vi "Load Default Modes v2.vi"(9 "SLM Param In":T1={"Error"={"status"=FALSE, "code"=0, "source"=""}, "References"={"Main VI"=refnum, "SLM VI"=refnum}, "Directories"={"Root Directory"=path "C:/Documents and Settings/tg273/My Documents/LabView VIs/Yale SLM/Yale v2/Mode Matrices", "Output Directory"=path "C:/Documents and Settings/tg273/My Documents/LabView VIs/Yale SLM/Yale v2/Mode Matrices"}, "Holo size"=504, "X pos"=-3, "Y pos"=-40, "Mode Coeffs"=[[2.0, 0.0], [3.0, 18.0], [4.0, 0.0], [11.0, 0.0], [22.0, 0.0], [37.0, 0.0], [5.0, 0.0], [6.0, 0.0], [7.0, 0.0], [8.0, 0.0], [9.0, 0.0], [10.0, 0.0]], "Wrap Value"=197, "Lambda (nm)"=750.0, "NA"=1.4, "Base Name"="", "Win Num"=2, "SLM SN"="0600535", "Holo Image Name"="0600535", "Matrix Name"="Unit Matrix.csv", "Mode Matrix"=array36x36[1296 elements], "Flatness"=array600x792[475200 elements], "STED Phase"=array504x504[254016 elements], "Ab Corr"=array504x504[254016 elements], "Holo Image"="remote image 00000000298188F4", "Holo Position"={-3.0, -40.0, 3840.0, 504.0}, "Apply Flatness\ncorr.?"=TRUE, "Max Wavelength (nm)"=750.0, "Min Wavelength (nm)"=750.0, "Vortex Rotation"=-3, "Top Hat Radius"=1.4, "SLM ID Num"="0600535", "Max Zernike Modes"=-3, "Screen Width"=2, "Ab Corr VI"={"AC VI Ref"=refnum, "# Modes"=2, "Mode Array"=[[4.0, 0.0, 0.0, 1.0, 0.0], [11.0, 0.75, 0.0, 1.0, 0.0], [22.0, 0.1, 0.0, 1.0, 0.0], [37.0, 0.0, 0.0, 1.0, 0.0], [7.0, 0.15, 0.0, 1.0, 0.0], [8.0, 0.1, 0.0, 1.0, 0.0], [5.0, 0.05, 0.0, 1.0, 0.0], [6.0, 0.0, 0.0, 1.0, 0.0], [9.0, 0.0, 0.0, 1.0, 0.0], [10.0, 0.0, 0.0, 1.0, 0.0], [2.0, 0.0, 0.0, 1.0, 0.0], [3.0, -18.3, 0.0, 1.0, 0.0]], "Apply Corr?"=TRUE, "Step Size"=0.3, "# Steps  "=11, "Resolution"=0.2, "FOV (um)"=12.0, "Metric Images"=[], "Metric Values"=[], "S"=[120.26, 128.5, 131.1, 136.15, 138.3, 148.05, 149.99, 150.02, 147.88, 152.65, 152.69, 150.56, 144.92, 143.08, 146.19, 140.15, 134.69, 125.47, 117.35, 108.32], "I"=[], "M"=[], "Coeff Steps"=[120.26, 128.5, 131.1, 136.15, 138.3, 148.05, 149.99, 150.02, 147.88, 152.65, 152.69, 150.56, 144.92, 143.08, 146.19, 140.15, 134.69, 125.47, 117.35, 108.32], "Mode Loop"={"Mode"=0, "Metric"=0, "Loop Index"=0}}} {"Vortex Rotation" format="%#_3g"; "Min Wavelength (nm)" format="%#_3g"; "Max Wavelength (nm)" format="%#_3g"; "Mode Matrix" format="%0.3f"; "Wrap Value" format="%#_3g"}) -> (1 "SLM Param Out":T1={"Error"={"status"=FALSE, "code"=0, "source"=""}, "References"={"Main VI"=refnum, "SLM VI"=refnum}, "Directories"={"Root Directory"=path "C:/Documents and Settings/tg273/My Documents/LabView VIs/Yale SLM/Yale v2/Mode Matrices", "Output Directory"=path "C:/Documents and Settings/tg273/My Documents/LabView VIs/Yale SLM/Yale v2/Mode Matrices"}, "Holo size"=504, "X pos"=-3, "Y pos"=-40, "Mode Coeffs"=[[2.0, 0.0], [3.0, 18.0], [4.0, 0.0], [11.0, 0.0], [22.0, 0.0], [37.0, 0.0], [5.0, 0.0], [6.0, 0.0], [7.0, 0.0], [8.0, 0.0], [9.0, 0.0], [10.0, 0.0]], "Wrap Value"=197, "Lambda (nm)"=750.0, "NA"=1.4, "Base Name"="", "Win Num"=2, "SLM SN"="0600535", "Holo Image Name"="0600535", "Matrix Name"="Unit Matrix.csv", "Mode Matrix"=array36x36[1296 elements], "Flatness"=array600x792[475200 elements], "STED Phase"=array504x504[254016 elements], "Ab Corr"=array504x504[254016 elements], "Holo Image"="remote image 00000000298188F4", "Holo Position"={-3.0, -40.0, 3840.0, 504.0}, "Apply Flatness\ncorr.?"=TRUE, "Max Wavelength (nm)"=750.0, "Min Wavelength (nm)"=750.0, "Vortex Rotation"=-3, "Top Hat Radius"=1.4, "SLM ID Num"="0600535", "Max Zernike Modes"=-3, "Screen Width"=2, "Ab Corr VI"={"AC VI Ref"=refnum, "# Modes"=2, "Mode Array"=[[4.0, 0.0, 0.0, 1.0, 0.0], [11.0, 0.75, 0.0, 1.0, 0.0], [22.0, 0.1, 0.0, 1.0, 0.0], [37.0, 0.0, 0.0, 1.0, 0.0], [7.0, 0.15, 0.0, 1.0, 0.0], [8.0, 0.1, 0.0, 1.0, 0.0], [5.0, 0.05, 0.0, 1.0, 0.0], [6.0, 0.0, 0.0, 1.0, 0.0], [9.0, 0.0, 0.0, 1.0, 0.0], [10.0, 0.0, 0.0, 1.0, 0.0], [2.0, 0.0, 0.0, 1.0, 0.0], [3.0, -18.3, 0.0, 1.0, 0.0]], "Apply Corr?"=TRUE, "Step Size"=0.3, "# Steps  "=11, "Resolution"=0.2, "FOV (um)"=12.0, "Metric Images"=[], "Metric Values"=[], "S"=[120.26, 128.5, 131.1, 136.15, 138.3, 148.05, 149.99, 150.02, 147.88, 152.65, 152.69, 150.56, 144.92, 143.08, 146.19, 140.15, 134.69, 125.47, 117.35, 108.32], "I"=[], "M"=[], "Coeff Steps"=[120.26, 128.5, 131.1, 136.15, 138.3, 148.05, 149.99, 150.02, 147.88, 152.65, 152.69, 150.56, 144.92, 143.08, 146.19, 140.15, 134.69, 125.47, 117.35, 108.32], "Mode Loop"={"Mode"=0, "Metric"=0, "Loop Index"=0}}} {"Vortex Rotation" format="%#_3g"; "Min Wavelength (nm)" format="%#_3g"; "Max Wavelength (nm)" format="%#_3g"; "Mode Matrix" format="%0.3f"; "Wrap Value" format="%#_3g"})   [LabVIEW 2014]
uses:
  TypeDefs/SLM Parameters.ctl
  <vilib>/vision/Image Controls.llb/IMAQ Image.ctl
  <vilib>/Utility/file.llb/Read From Spreadsheet File (DBL).vi
types:
  T1 = typedef "SLM Parameters.ctl" = cluster{"Error":errorcluster, "References":cluster{"Main VI":refnum<vi>, "SLM VI":refnum<vi>}, "Directories":cluster{"Root Directory":path, "Output Directory":path}, "Holo size":u16, "X pos":i16, "Y pos":i16, "Mode Coeffs":dbl[][], "Wrap Value":i32, "Lambda (nm)":dbl, "NA":dbl, "Base Name":string, "Win Num":i32, "SLM SN":string, "Holo Image Name":string, "Matrix Name":string, "Mode Matrix":dbl[][], "Flatness":u8[][], "STED Phase":dbl[][], "Ab Corr":dbl[][], "Holo Image":T2, "Holo Position":cluster{dbl, dbl, dbl, dbl}, "Apply Flatness\ncorr.?":bool, "Max Wavelength (nm)":dbl, "Min Wavelength (nm)":dbl, "Vortex Rotation":i16, "Top Hat Radius":dbl, "SLM ID Num":string, "Max Zernike Modes":i16, "Screen Width":i32, "Ab Corr VI":cluster{"AC VI Ref":refnum<vi>, "# Modes":i32, "Mode Array":dbl[][], "Apply Corr?":bool, "Step Size":dbl, "# Steps  ":u16, "Resolution":dbl, "FOV (um)":dbl, "Metric Images":dbl[][][][], "Metric Values":dbl[][], "S":dbl[], "I":dbl[], "M":dbl[], "Coeff Steps":dbl[], "Mode Loop":cluster{"Mode":i8, "Metric":i8, "Loop Index":i8}}}
  T2 = typedef "IMAQ Image.ctl" = refnum<image>
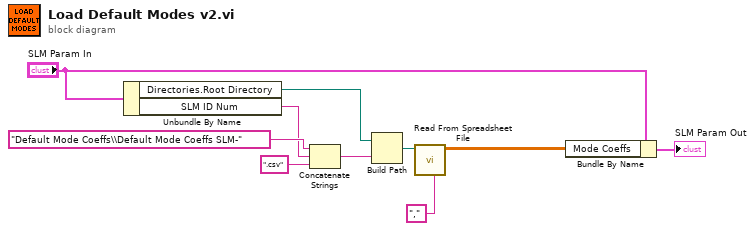
[diagram p0: block diagram]
diagram:
  n1 = Unbundle By Name("SLM Param In") -> ("Directories.Root Directory"=w9:path, "SLM ID Num"=w5:string)
  n2 = Concatenate Strings("Default Mode Coeffs\\Default Mode Coeffs SLM-" ("string"), w5, ".csv" ("string")) -> (w8:string)
  n3 = Build Path(base path=w9, name or relative path=w8) -> (appended path=w4:path)
  n4 = call-poly <vilib>:"Read From Spreadsheet File.vi"("delimiter (\\t)"="," ("delimiter (\\t)"), "file path (dialog if empty)"=w4) -> ("all rows"=w1:dbl[][])  [unwired: 3 in, 6 out]
  n5 = Bundle By Name(cluster="SLM Param In", "Mode Coeffs"=w1) -> (→"SLM Param Out":T1)
